vi "Dresden R2R Sputter 03.02.2018 IY24.vi"() -> ()   [LabVIEW 2009] (continued)
                                n28242 = case shown="True" w33302 {
                                frame #0 {
                                }
                                frame #1 {
                                n28243 = local write "Semi"(TRUE ("Semi")) -> ()
                                n28244 = local write "Error Message"("Coating Process  \nwas cancelled.\nPlease check \nBG-BV connection." ("Error Message")) -> ()
                                }
                                }
                                n28245 = local read "Ch4_Cc_on_off_di"() -> (w33301:bool)
                                n28246 = case shown="True" w33301 {
                                tunnel: [TRUE FALSE] -> w33300
                                frame #0 {
                                }
                                frame #1 {
                                n28247 = local write "Ch4_Cc_on_off_do"(FALSE ("Ch1_WFC_do")) -> ()
                                n28248 = Wait Until Next ms Multiple(millisecond multiple=u32 200) -> ()  [unwired: 1 out]
                                }
                                }
                                n28249 = local read "Semi"() -> (w33299:bool)
                                n28250 = Or(x=w33300, y=w33299) -> (x .or. y?=w33298:bool)
                                }
                                }
                                frame #1 {
                                }
                                }
                                }
                                frame #1 {
                                n28251 = local read "Semi"() -> (w33311:bool)
                                n28252 = case shown="False" w33311 {
                                frame #0 {
                                n28253 = local write "SDC1 3"(TRUE ("SDC1 3")) -> ()
                                n28254 = Wait (ms)(milliseconds to wait=u32 1000) -> ()  [unwired: 1 out]
                                }
                                frame #1 {
                                }
                                }
                                }
                                }
                                }
                                frame #6 {
                                # "PC-BV CLOSE"
                                n28255 = stacked-sequence {
                                frame #0 {
                                n28256 = local read "Semi"() -> (w33314:bool)
                                n28257 = case shown="False" w33314 {
                                frame #0 {
                                n28258 = stacked-sequence {
                                frame #0 {
                                n28259 = local read "Semi"() -> (w33315:bool)
                                n28260 = case shown="False" w33315 {
                                frame #0 {
                                n28261 = local write "Pc_bv4_auto_close"(TRUE ("Tp1_auto_start")) -> ()
                                }
                                frame #1 {
                                }
                                }
                                }
                                frame #1 {
                                n28262 = local read "Semi"() -> (w33317:bool)
                                n28263 = case shown="False" w33317 {
                                frame #0 {
                                n28264 = Wait (ms)(milliseconds to wait=u32 1000) -> ()  [unwired: 1 out]
                                }
                                frame #1 {
                                }
                                }
                                }
                                frame #2 {
                                n28265 = local read "Semi"() -> (w33319:bool)
                                n28266 = case shown="False" w33319 {
                                frame #0 {
                                n28267 = while {
                                i -> [w33325]
                                stop <- w33321 stop-if-true
                                n28268 = local read "Pc_bv_closed_ch4"() -> (w33323:bool)
                                n28269 = Greater?(x=w33325, y=120) -> (0:w33324:bool)
                                n28270 = local read "Semi"() -> (w33322:bool)
                                n28271 = Compound Arithmetic op=OR(w33322, w33323, w33324) -> (w33321:bool)
                                n28272 = Wait (ms)(milliseconds to wait=u32 500) -> ()  [unwired: 1 out]
                                }
                                }
                                frame #1 {
                                }
                                }
                                }
                                frame #3 {
                                n28273 = local read "Semi"() -> (w33327:bool)
                                n28274 = case shown="False" w33327 {
                                frame #0 {
                                n28275 = local read "Pc_bv_closed_ch4"() -> (w33328:bool)
                                n28276 = case shown="False" w33328 {
                                frame #0 {
                                n28277 = local write "Pc_bv4_auto_close"(TRUE ("Pc_bv1_auto_open")) -> ()
                                }
                                frame #1 {
                                }
                                }
                                }
                                frame #1 {
                                }
                                }
                                }
                                frame #4 {
                                n28278 = local read "Semi"() -> (w33330:bool)
                                n28279 = case shown="False" w33330 {
                                frame #0 {
                                n28280 = local read "Pc_bv_closed_ch4"() -> (w33331:bool)
                                n28281 = case shown="False" w33331 {
                                frame #0 {
                                n28282 = Wait (ms)(milliseconds to wait=u32 1000) -> ()  [unwired: 1 out]
                                }
                                frame #1 {
                                }
                                }
                                }
                                frame #1 {
                                }
                                }
                                }
                                frame #5 {
                                n28283 = local read "Semi"() -> (w33333:bool)
                                n28284 = case shown="False" w33333 {
                                frame #0 {
                                n28285 = while {
                                i -> [w33339]
                                stop <- w33335 stop-if-true
                                n28286 = local read "Pc_bv_closed_ch4"() -> (w33337:bool)
                                n28287 = Greater?(x=w33339, y=120) -> (0:w33338:bool)
                                n28288 = local read "Semi"() -> (w33336:bool)
                                n28289 = Compound Arithmetic op=OR(w33336, w33337, w33338) -> (w33335:bool)
                                n28290 = Wait (ms)(milliseconds to wait=u32 500) -> ()  [unwired: 1 out]
                                }
                                }
                                frame #1 {
                                }
                                }
                                }
                                frame #6 {
                                n28291 = local read "Semi"() -> (w33341:bool)
                                n28292 = case shown="False" w33341 {
                                frame #0 {
                                n28293 = local read "Pc_bv_closed_ch4"() -> (w33342:bool)
                                n28294 = case shown="False" w33342 {
                                frame #0 {
                                n28295 = local write "Error Message"("Start up process  cancelled\nbecause  PC-BV not closed.\nPlease check PC-BV1 connections." ("Error Message")) -> ()
                                n28296 = Wait (ms)(milliseconds to wait=u32 1000) -> ()  [unwired: 1 out]
                                }
                                frame #1 {
                                }
                                }
                                }
                                frame #1 {
                                }
                                }
                                }
                                }
                                }
                                frame #1 {
                                }
                                }
                                }
                                frame #1 {
                                n28297 = local read "Semi"() -> (w33345:bool)
                                n28298 = case shown="False" w33345 {
                                frame #0 {
                                n28299 = local write "SDC1 5"(TRUE ("SDC1 5")) -> ()
                                n28300 = Wait (ms)(milliseconds to wait=u32 1000) -> ()  [unwired: 1 out]
                                }
                                frame #1 {
                                }
                                }
                                }
                                }
                                }
                                frame #7 {
                                # "SOV-AR OPEN"
                                n28301 = stacked-sequence {
                                frame #0 {
                                n28302 = local read "Semi"() -> (w33348:bool)
                                n28303 = case shown="False" w33348 {
                                frame #0 {
                                n28304 = while {
                                i -> [w33354]
                                stop <- w33349 stop-if-true
                                n28305 = Greater?(x=w33354, y=50) -> (0:w33353:bool)
                                n28306 = case shown="True" w33353 {
                                frame #0 {
                                }
                                frame #1 {
                                n28307 = local write "Semi"(TRUE ("Semi")) -> ()
                                n28308 = local write "Error Message"("Coating Process  \nwas cancelled.\nPlease check \nSOV-Ar connection." ("Error Message")) -> ()
                                }
                                }
                                n28309 = local read "Ch4_Sov_Ar_di"() -> (w33352:bool)
                                n28310 = case shown="False" w33352 {
                                tunnel: [FALSE TRUE] -> w33351
                                frame #0 {
                                n28311 = local write "Ch4_Sov_Ar_do"(TRUE ("Ch1_WFC_do")) -> ()
                                n28312 = Wait Until Next ms Multiple(millisecond multiple=u32 200) -> ()  [unwired: 1 out]
                                }
                                frame #1 {
                                }
                                }
                                n28313 = local read "Semi"() -> (w33350:bool)
                                n28314 = Or(x=w33351, y=w33350) -> (x .or. y?=w33349:bool)
                                }
                                }
                                frame #1 {
                                }
                                }
                                }
                                frame #1 {
                                n28315 = local read "Semi"() -> (w33362:bool)
                                n28316 = case shown="False" w33362 {
                                frame #0 {
                                n28317 = while {
                                i -> [w33367]
                                stop <- w33365 stop-if-true
                                n28318 = Greater?(x=w33367, y=5) -> (0:w33363:bool)
                                n28319 = Wait Until Next ms Multiple(millisecond multiple=u32 1000) -> ()  [unwired: 1 out]
                                n28320 = local read "Semi"() -> (w33366:bool)
                                n28321 = Or(x=w33363, y=w33366) -> (x .or. y?=w33365:bool)
                                }
                                }
                                frame #1 {
                                }
                                }
                                }
                                frame #2 {
                                n28322 = local read "Semi"() -> (w33369:bool)
                                n28323 = case shown="False" w33369 {
                                frame #0 {
                                n28324 = local write "SDC1 6"(TRUE ("SDC1 6")) -> ()
                                n28325 = Wait (ms)(milliseconds to wait=u32 1000) -> ()  [unwired: 1 out]
                                }
                                frame #1 {
                                }
                                }
                                }
                                }
                                }
                                frame #8 {
                                # "CHECK CHAMBER PRESSURE"
                                n28326 = stacked-sequence {
                                frame #0 {
                                n28327 = local read "Semi"() -> (w33372:bool)
                                n28328 = case shown="False" w33372 {
                                frame #0 {
                                n28329 = while {
                                i -> [w33380]
                                stop <- w33374 stop-if-true
                                n28330 = Greater?(x=w33380, y=300) -> (0:w33379:bool)
                                n28331 = case shown="True" w33379 {
                                frame #0 {
                                }
                                frame #1 {
                                n28332 = local write "Semi"(TRUE ("Semi")) -> ()
                                n28333 = local write "Error Message"("Coating Process cancelled.\nPlease check chamber \nconnections." ("Error Message")) -> ()
                                }
                                }
                                n28334 = local read "Ch_pg_press_ch4_gui"() -> (w33373:dbl)
                                n28335 = Greater Or Equal?(x=w33373, y=0.9 ("CHAMBER PRESSURE 4")) -> (x >= y?=w33377:bool)
                                n28336 = case shown="True" w33377 {
                                tunnel: [TRUE FALSE] -> w33376
                                frame #0 {
                                }
                                frame #1 {
                                n28337 = Wait Until Next ms Multiple(millisecond multiple=u32 200) -> ()  [unwired: 1 out]
                                }
                                }
                                n28338 = local read "Semi"() -> (w33375:bool)
                                n28339 = Or(x=w33376, y=w33375) -> (x .or. y?=w33374:bool)
                                }
                                }
                                frame #1 {
                                }
                                }
                                }
                                frame #1 {
                                n28340 = local read "Semi"() -> (w33387:bool)
                                n28341 = case shown="False" w33387 {
                                frame #0 {
                                n28342 = Wait (ms)(milliseconds to wait=u32 1000) -> ()  [unwired: 1 out]
                                n28343 = local write "SDC1 8"(TRUE ("SDC1 8")) -> ()
                                }
                                frame #1 {
                                }
                                }
                                }
                                }
                                }
                                frame #9 {
                                # "PC-BV OPEN"
                                n28344 = stacked-sequence {
                                frame #0 {
                                n28345 = local read "Semi"() -> (w33390:bool)
                                n28346 = case shown="False" w33390 {
                                frame #0 {
                                n28347 = stacked-sequence {
                                frame #0 {
                                n28348 = local read "Semi"() -> (w33391:bool)
                                n28349 = case shown="False" w33391 {
                                frame #0 {
                                n28350 = local write "Pc_bv4_auto_open"(TRUE ("Tp1_auto_start")) -> ()
                                }
                                frame #1 {
                                }
                                }
                                }
                                frame #1 {
                                n28351 = local read "Semi"() -> (w33393:bool)
                                n28352 = case shown="False" w33393 {
                                frame #0 {
                                n28353 = Wait (ms)(milliseconds to wait=u32 1000) -> ()  [unwired: 1 out]
                                }
                                frame #1 {
                                }
                                }
                                }
                                frame #2 {
                                n28354 = local read "Semi"() -> (w33395:bool)
                                n28355 = case shown="False" w33395 {
                                frame #0 {
                                n28356 = while {
                                i -> [w33401]
                                stop <- w33397 stop-if-true
                                n28357 = local read "Pc_bv_opened_ch4"() -> (w33399:bool)
                                n28358 = Greater?(x=w33401, y=120) -> (0:w33400:bool)
                                n28359 = local read "Semi"() -> (w33398:bool)
                                n28360 = Compound Arithmetic op=OR(w33398, w33399, w33400) -> (w33397:bool)
                                n28361 = Wait (ms)(milliseconds to wait=u32 500) -> ()  [unwired: 1 out]
                                }
                                }
                                frame #1 {
                                }
                                }
                                }
                                frame #3 {
                                n28362 = local read "Semi"() -> (w33403:bool)
                                n28363 = case shown="False" w33403 {
                                frame #0 {
                                n28364 = local read "Pc_bv_opened_ch4"() -> (w33404:bool)
                                n28365 = case shown="False" w33404 {
                                frame #0 {
                                n28366 = local write "Pc_bv4_auto_open"(TRUE ("Pc_bv1_auto_open")) -> ()
                                }
                                frame #1 {
                                }
                                }
                                }
                                frame #1 {
                                }
                                }
                                }
                                frame #4 {
                                n28367 = local read "Semi"() -> (w33406:bool)
                                n28368 = case shown="False" w33406 {
                                frame #0 {
                                n28369 = local read "Pc_bv_opened_ch4"() -> (w33407:bool)
                                n28370 = case shown="False" w33407 {
                                frame #0 {
                                n28371 = Wait (ms)(milliseconds to wait=u32 1000) -> ()  [unwired: 1 out]
                                }
                                frame #1 {
                                }
                                }
                                }
                                frame #1 {
                                }
                                }
                                }
                                frame #5 {
                                n28372 = local read "Semi"() -> (w33409:bool)
                                n28373 = case shown="False" w33409 {
                                frame #0 {
                                n28374 = while {
                                i -> [w33415]
                                stop <- w33411 stop-if-true
                                n28375 = local read "Pc_bv_opened_ch4"() -> (w33413:bool)
                                n28376 = Greater?(x=w33415, y=120) -> (0:w33414:bool)
                                n28377 = local read "Semi"() -> (w33412:bool)
                                n28378 = Compound Arithmetic op=OR(w33412, w33413, w33414) -> (w33411:bool)
                                n28379 = Wait (ms)(milliseconds to wait=u32 500) -> ()  [unwired: 1 out]
                                }
                                }
                                frame #1 {
                                }
                                }
                                }
                                frame #6 {
                                n28380 = local read "Semi"() -> (w33417:bool)
                                n28381 = case shown="False" w33417 {
                                frame #0 {
                                n28382 = local read "Pc_bv_opened_ch4"() -> (w33418:bool)
                                n28383 = case shown="False" w33418 {
                                frame #0 {
                                n28384 = local write "Error Message"("Start up process  cancelled\nbecause  PC-BV not opened.\nPlease check PC-BV1 connections." ("Error Message")) -> ()
                                n28385 = Wait (ms)(milliseconds to wait=u32 1000) -> ()  [unwired: 1 out]
                                }
                                frame #1 {
                                }
                                }
                                }
                                frame #1 {
                                }
                                }
                                }
                                }
                                }
                                frame #1 {
                                }
                                }
                                }
                                frame #1 {
                                n28386 = local read "Semi"() -> (w33421:bool)
                                n28387 = case shown="False" w33421 {
                                frame #0 {
                                n28388 = Wait (ms)(milliseconds to wait=u32 1000) -> ()  [unwired: 1 out]
                                n28389 = local write "SDC1 7"(TRUE ("SDC1 7")) -> ()
                                }
                                frame #1 {
                                }
                                }
                                }
                                }
                                }
                                frame #10 {
                                # "CC OPEN"
                                n28390 = stacked-sequence {
                                frame #0 {
                                n28391 = local read "Semi"() -> (w33424:bool)
                                n28392 = case shown="False" w33424 {
                                frame #0 {
                                n28393 = while {
                                i -> [w33430]
                                stop <- w33425 stop-if-true
                                n28394 = Greater?(x=w33430, y=50) -> (0:w33429:bool)
                                n28395 = case shown="True" w33429 {
                                frame #0 {
                                }
                                frame #1 {
                                n28396 = local write "Semi"(TRUE ("Semi")) -> ()
                                n28397 = local write "Error Message"("Coating Process  \nwas cancelled.\nPlease check \nBG-BV connection." ("Error Message")) -> ()
                                }
                                }
                                n28398 = local read "Ch4_Cc_on_off_di"() -> (w33428:bool)
                                n28399 = case shown="False" w33428 {
                                tunnel: [FALSE TRUE] -> w33427
                                frame #0 {
                                n28400 = local write "Ch4_Cc_on_off_do"(TRUE ("Ch1_WFC_do")) -> ()
                                n28401 = Wait Until Next ms Multiple(millisecond multiple=u32 200) -> ()  [unwired: 1 out]
                                }
                                frame #1 {
                                }
                                }
                                n28402 = local read "Semi"() -> (w33426:bool)
                                n28403 = Or(x=w33427, y=w33426) -> (x .or. y?=w33425:bool)
                                }
                                }
                                frame #1 {
                                }
                                }
                                }
                                frame #1 {
                                n28404 = local read "Semi"() -> (w33438:bool)
                                n28405 = case shown="False" w33438 {
                                frame #0 {
                                n28406 = while {
                                i -> [w33443]
                                stop <- w33441 stop-if-true
                                n28407 = Greater?(x=w33443, y=30) -> (0:w33439:bool)
                                n28408 = Wait Until Next ms Multiple(millisecond multiple=u32 1000) -> ()  [unwired: 1 out]
                                n28409 = local read "Semi"() -> (w33442:bool)
                                n28410 = Or(x=w33439, y=w33442) -> (x .or. y?=w33441:bool)
                                }
                                }
                                frame #1 {
                                }
                                }
                                }
                                frame #2 {
                                n28411 = local read "Semi"() -> (w33445:bool)
                                n28412 = case shown="False" w33445 {
                                frame #0 {
                                n28413 = Wait (ms)(milliseconds to wait=u32 1000) -> ()  [unwired: 1 out]
                                n28414 = local write "SDC1 7b"(TRUE ("SDC1 3")) -> ()
                                }
                                frame #1 {
                                }
                                }
                                }
                                }
                                }
                                frame #11 {
                                # "CHECK CHAMBER PRESSURE"
                                n28415 = stacked-sequence {
                                frame #0 {
                                n28416 = local read "Semi"() -> (w33448:bool)
                                n28417 = case shown="False" w33448 {
                                frame #0 {
                                n28418 = while {
                                i -> [w33456]
                                stop <- w33450 stop-if-true
                                n28419 = Greater?(x=w33456, y=300) -> (0:w33455:bool)
                                n28420 = case shown="True" w33455 {
                                frame #0 {
                                }
                                frame #1 {
                                n28421 = local write "Semi"(TRUE ("Semi")) -> ()
                                n28422 = local write "Error Message"("Coating Process cancelled.\nPlease check chamber \nconnections." ("Error Message")) -> ()
                                }
                                }
                                n28423 = local read "Ch_CC_press_ch4_2"() -> (w33449:dbl)
                                n28424 = Greater Or Equal?(x=w33449, y=5e-05 ("CHAMBER PRESSURE 5")) -> (x >= y?=w33453:bool)
                                n28425 = case shown="True" w33453 {
                                tunnel: [TRUE FALSE] -> w33452
                                frame #0 {
                                }
                                frame #1 {
                                n28426 = Wait Until Next ms Multiple(millisecond multiple=u32 200) -> ()  [unwired: 1 out]
                                }
                                }
                                n28427 = local read "Semi"() -> (w33451:bool)
                                n28428 = Or(x=w33452, y=w33451) -> (x .or. y?=w33450:bool)
                                }
                                }
                                frame #1 {
                                }
                                }
                                }
                                frame #1 {
                                n28429 = local read "Semi"() -> (w33463:bool)
                                n28430 = case shown="False" w33463 {
                                frame #0 {
                                n28431 = Wait (ms)(milliseconds to wait=u32 1000) -> ()  [unwired: 1 out]
                                n28432 = local write "SDC1 10"(TRUE ("SDC1 10")) -> ()
                                }
                                frame #1 {
                                }
                                }
                                }
                                }
                                }
                                frame #12 {
                                # "CC CLOSE"
                                n28433 = stacked-sequence {
                                frame #0 {
                                n28434 = local read "Semi"() -> (w33466:bool)
                                n28435 = case shown="False" w33466 {
                                frame #0 {
                                n28436 = while {
                                i -> [w33472]
                                stop <- w33467 stop-if-true
                                n28437 = Greater?(x=w33472, y=50) -> (0:w33471:bool)
                                n28438 = case shown="True" w33471 {
                                frame #0 {
                                }
                                frame #1 {
                                n28439 = local write "Semi"(TRUE ("Semi")) -> ()
                                n28440 = local write "Error Message"("Coating Process  \nwas cancelled.\nPlease check \nBG-BV connection." ("Error Message")) -> ()
                                }
                                }
                                n28441 = local read "Ch4_Cc_on_off_di"() -> (w33470:bool)
                                n28442 = case shown="True" w33470 {
                                tunnel: [TRUE FALSE] -> w33469
                                frame #0 {
                                }
                                frame #1 {
                                n28443 = local write "Ch4_Cc_on_off_do"(FALSE ("Ch1_WFC_do")) -> ()
                                n28444 = Wait Until Next ms Multiple(millisecond multiple=u32 200) -> ()  [unwired: 1 out]
                                }
                                }
                                n28445 = local read "Semi"() -> (w33468:bool)
                                n28446 = Or(x=w33469, y=w33468) -> (x .or. y?=w33467:bool)
                                }
                                }
                                frame #1 {
                                }
                                }
                                }
                                frame #1 {
                                n28447 = local read "Semi"() -> (w33480:bool)
                                n28448 = case shown="False" w33480 {
                                frame #0 {
                                n28449 = local write "SDC1 10b"(TRUE ("SDC1 3")) -> ()
                                n28450 = Wait (ms)(milliseconds to wait=u32 1000) -> ()  [unwired: 1 out]
                                }
                                frame #1 {
                                }
                                }
                                }
                                }
                                }
                                frame #13 {
                                # "SET Ar FLOW"
                                n28451 = local read "R_Web_selection"() -> (w33483:enum32{"Web", "Other"})
                                n28452 = case shown="\"Other\"" w33483 {
                                frame #0 {
                                }
                                frame #1 {
                                n28453 = stacked-sequence {
                                frame #0 {
                                n28454 = local read "Semi"() -> (w33484:bool)
                                n28455 = case shown="False" w33484 {
                                frame #0 {
                                n28456 = stacked-sequence {
                                frame #0 {
                                n28457 = local read "Semi"() -> (w33485:bool)
                                n28458 = case shown="False" w33485 {
                                frame #0 {
                                n28459 = local read "R Argon Flow sccm"() -> (w33486:dbl)
                                n28460 = local write "Ar_sccm3_4"(w33486) -> ()
                                }
                                frame #1 {
                                }
                                }
                                }
                                frame #1 {
                                n28461 = local read "Semi"() -> (w33487:bool)
                                n28462 = case shown="False" w33487 {
                                frame #0 {
                                n28463 = local write "Mfc2_Ar _3_4_set"(TRUE ("Mfc_Ar _1_2_set")) -> ()
                                }
                                frame #1 {
                                }
                                }
                                }
                                frame #2 {
                                n28464 = local read "Semi"() -> (w33489:bool)
                                n28465 = case shown="False" w33489 {
                                frame #0 {
                                n28466 = while {
                                i -> [w33492]
                                stop <- w33494 stop-if-true
                                n28467 = Greater?(x=w33492, y=50) -> (0:w33491:bool)
                                n28468 = local read "Semi"() -> (w33490:bool)
                                n28469 = Or(x=w33490, y=w33491) -> (x .or. y?=w33494:bool)
                                }
                                }
                                frame #1 {
                                }
                                }
                                }
                                frame #3 {
                                n28470 = local read "Semi"() -> (w33495:bool)
                                n28471 = case shown="False" w33495 {
                                frame #0 {
                                n28472 = local read "Ar_sccm_act 2"() -> (w33496:dbl)
                                n28473 = Greater?(x=w33496, y=1) -> (0:w33497:bool)
                                n28474 = case shown="False" w33497 {
                                frame #0 {
                                n28475 = local read "R Argon Flow sccm"() -> (w33499:dbl)
                                n28476 = local write "Ar_sccm3_4"(w33499) -> ()
                                }
                                frame #1 {
                                }
                                }
                                }
                                frame #1 {
                                }
                                }
                                }
                                frame #4 {
                                n28477 = local read "Semi"() -> (w33500:bool)
                                n28478 = case shown="False" w33500 {
                                frame #0 {
                                n28479 = local read "Ar_sccm_act 2"() -> (w33501:dbl)
                                n28480 = Greater?(x=w33501, y=1) -> (0:w33502:bool)
                                n28481 = case shown="False" w33502 {
                                frame #0 {
                                n28482 = while {
                                i -> [w33505]
                                stop <- w33509 stop-if-true
                                n28483 = Greater?(x=w33505, y=50) -> (0:w33504:bool)
                                n28484 = local read "Semi"() -> (w33508:bool)
                                n28485 = case shown="False" w33508 {
                                tunnel: [FALSE TRUE] -> w33507
                                frame #0 {
                                n28486 = Wait Until Next ms Multiple(millisecond multiple=u32 200) -> ()  [unwired: 1 out]
                                }
                                frame #1 {
                                }
                                }
                                n28487 = Or(x=w33507, y=w33504) -> (x .or. y?=w33509:bool)
                                }
                                }
                                frame #1 {
                                }
                                }
                                }
                                frame #1 {
                                }
                                }
                                }
                                frame #5 {
                                n28488 = local read "Semi"() -> (w33513:bool)
                                n28489 = case shown="False" w33513 {
                                frame #0 {
                                n28490 = local read "Ar_sccm_act 2"() -> (w33514:dbl)
                                n28491 = Greater?(x=w33514, y=1) -> (0:w33515:bool)
                                n28492 = case shown="False" w33515 {
                                frame #0 {
                                n28493 = local write "Semi"(TRUE ("Semi")) -> ()
                                n28494 = local write "Error Message"("Coating process cancelled.\nPlease check connections." ("Error Message")) -> ()
                                }
                                frame #1 {
                                }
                                }
                                }
                                frame #1 {
                                }
                                }
                                }
                                }
                                }
                                frame #1 {
                                }
                                }
                                }
                                frame #1 {
                                n28495 = local read "Semi"() -> (w33519:bool)
                                n28496 = case shown="False" w33519 {
                                frame #0 {
                                n28497 = local write "SDC1 11"(TRUE ("SDC1 11")) -> ()
                                n28498 = Wait (ms)(milliseconds to wait=u32 1000) -> ()  [unwired: 1 out]
                                }
                                frame #1 {
                                }
                                }
                                }
                                }
                                }
                                }
                                }
                                frame #14 {
                                # "Set  Pressure"
                                n28499 = local read "R_Web_selection"() -> (w33522:enum32{"Web", "Other"})
                                n28500 = case shown="\"Other\"" w33522 {
                                frame #0 {
                                }
                                frame #1 {
                                n28501 = stacked-sequence {
                                frame #0 {
                                n28502 = local read "Semi"() -> (w33523:bool)
                                n28503 = case shown="False" w33523 {
                                frame #0 {
                                n28504 = stacked-sequence {
                                frame #0 {
                                n28505 = local read "Semi"() -> (w33524:bool)
                                n28506 = case shown="False" w33524 {
                                frame #0 {
                                n28507 = local read "R Set Pressure mtorr"() -> (w33525:dbl)
                                n28508 = local write "Set_pressure_value 4"(w33525) -> ()
                                }
                                frame #1 {
                                }
                                }
                                }
                                frame #1 {
                                n28509 = local read "Semi"() -> (w33526:bool)
                                n28510 = case shown="False" w33526 {
                                frame #0 {
                                n28511 = Wait (ms)(milliseconds to wait=u32 1000) -> ()  [unwired: 1 out]
                                }
                                frame #1 {
                                }
                                }
                                }
                                frame #2 {
                                n28512 = local read "Semi"() -> (w33528:bool)
                                n28513 = case shown="False" w33528 {
                                frame #0 {
                                n28514 = local write "Pc_bv4_auto_set_pressure"(TRUE ("Pc_bv1_auto_set_pressure")) -> ()
                                }
                                frame #1 {
                                }
                                }
                                }
                                frame #3 {
                                n28515 = local read "Semi"() -> (w33530:bool)
                                n28516 = case shown="False" w33530 {
                                frame #0 {
                                n28517 = while {
                                i -> [w33541]
                                stop <- w33533 stop-if-true
                                n28518 = Greater?(x=w33541, y=300) -> (0:w33535:bool)
                                n28519 = local read "Set_pressure_value 4"() -> (w33531:dbl)
                                n28520 = Add(x=1.0, y=w33531) -> (x+y=w33537:dbl)
                                n28521 = Subtract(x=w33531, y=1.0) -> (x-y=w33538:dbl)
                                n28522 = local read "Pressure 4"() -> (w33532:i32)
                                n28523 = In Range and Coerce(upper limit=w33537, x=w33532, lower limit=w33538) -> (In Range?=w33536:bool)  [unwired: 1 out]
                                n28524 = case shown="False" w33536 {
                                tunnel: [FALSE TRUE] -> w33534
                                frame #0 {
                                n28525 = Wait Until Next ms Multiple(millisecond multiple=u32 200) -> ()  [unwired: 1 out]
                                }
                                frame #1 {
                                }
                                }
                                n28526 = Or(x=w33534, y=w33535) -> (x .or. y?=w33533:bool)
                                }
                                }
                                frame #1 {
                                }
                                }
                                }
                                frame #4 {
                                n28527 = local read "Semi"() -> (w33546:bool)
                                n28528 = case shown="False" w33546 {
                                frame #0 {
                                n28529 = local read "Set_pressure_value 4"() -> (w33548:dbl)
                                n28530 = Add(x=1.0, y=w33548) -> (x+y=w33550:dbl)
                                n28531 = Subtract(x=w33548, y=1.0) -> (x-y=w33551:dbl)
                                n28532 = local read "Pressure 4"() -> (w33547:i32)
                                n28533 = In Range and Coerce(upper limit=w33550, x=w33547, lower limit=w33551) -> (In Range?=w33549:bool)  [unwired: 1 out]